vi "FFT.vi"() -> ()   [LabVIEW 2021]
uses:
  ark_all/arkady-arxiv/cursor winow sygnal plot.ctl
  ark_all/arkady-arxiv/show-win- control.ctl
  ark_all/arkady-arxiv/cursor window action.ctl
  <vilib>/measure/maspectr.llb/FFT Power Spectrum for N Chan.vi
  <vilib>/measure/NI_MAPro.lvlib
panel:
  out "time (sec)":dbl=0.04508427
  in  "offset factor":dbl=100.0
  out "win (sec)":dbl=0.010354
  in  "digitization freq":dbl=3000000.0
  in  "win 2":T1={"cen (Hz)"=32754.180483243686, "win (Hz)"=308.86311527720136, "left (Hz)"=32599.748925605087, "right (Hz)"=32908.61204088229} {"right (Hz)" format="%#_3p"}
  out "dt (sec)":dbl=3.3e-07
  in  "cursor window":T2={"left"=0.04139793333333315, "right "=0.05175193333333315, "center"=0.04657493333333315, "window"=0.010354, "cursors"=[0, 1, 2], "relative"=0, "absolute"=0, "fixed vertical offset"=0.0, "vertical offset"=0.0, "skew"=0.0, "default window frac"=0.1, "kind"=enum."symmetric", "skew.left"=0.5, "skew.right"=0.5, "wing order"=enum."back", "Plot ref Syg"=refnum}
  in  "run":bool
  in  "Data window":T3={"Start"=124194, "Length"=31062, "Channel numbers"=[0], "Cannel names"=["freq", ""], "Group name"="p"}
  out "Signal graph":waveform(dbl)[](graph)=[{"t0"=timestamp(-0.009969989999999984 s since 1904-01-01), "dt"=3.3e-07, "Y"=array[333333 elements], "attributes"=variant("Configuration"=variant(string "[Configuration]\nConfiguration.Post-trigger delay = \"-0.010000000000\"\nConfiguration.Post-trigger duration = \"0.10000000000\"\nConfiguration.Rate = \"3030303.0303\"\nConfiguration.Ranges = \"<size(s)=5> 10.000000000 10.000000000 10.000000000 1.0000000000 1.0000000000\"\nConfiguration.Re-name channels.<size(s)> = \"5\"\nConfiguration.Re-name channels 0 = \"Idot\"\nConfiguration.Re-name channels 1 = \"Bdot\"\nConfiguration.Re-name channels 2 = \"Bproj\"\nConfiguration.Re-name channels 3 = \"freq\"\nConfiguration.Re-name channels 4 = \"drive\"\nConfiguration.Active channels = \"0,1,2,5,6\"\nConfiguration.External\\nclock = \"FALSE\"\nConfiguration.Monitor time\\nconstant = \"1.0000000000\"\nConfiguration.Sync = \"TRUE\"\nConfiguration.Lock-in input channel phases = \"<size(s)=0> \"\nConfiguration.Output channels configuration.<size(s)> = \"0\""), "NI_ChannelName"=variant(string "freq"))}]
  in  "Preserve old data":bool=TRUE
  out "FFT Graph":cluster{"f0":dbl, "df":dbl, "magnitude":dbl[]}[](graph)=[{"f0"=0.0, "df"=97.55659746001642, "magnitude"=array[15531 elements]}, {"f0"=0.0, "df"=97.55659746001642, "magnitude"=array[15531 elements]}, {"f0"=0.0, "df"=97.55659746001642, "magnitude"=array[15531 elements]}, {"f0"=0.0, "df"=97.55659746001642, "magnitude"=array[15531 elements]}, {"f0"=0.0, "df"=97.55659746001642, "magnitude"=array[15531 elements]}, {"f0"=0.0, "df"=97.55659746001642, "magnitude"=array[15531 elements]}, {"f0"=0.0, "df"=97.55659746001642, "magnitude"=array[15531 elements]}, {"f0"=0.0, "df"=97.55659746001642, "magnitude"=array[15531 elements]}, {"f0"=0.0, "df"=97.55659746001642, "magnitude"=array[15531 elements]}, {"f0"=0.0, "df"=97.55659746001642, "magnitude"=array[15531 elements]}, {"f0"=0.0, "df"=97.55659746001642, "magnitude"=array[15531 elements]}, {"f0"=0.0, "df"=97.55659746001642, "magnitude"=array[15531 elements]}, {"f0"=0.0, "df"=97.55659746001642, "magnitude"=array[15531 elements]}, {"f0"=0.0, "df"=97.55659746001642, "magnitude"=array[15531 elements]}, {"f0"=0.0, "df"=97.55659746001642, "magnitude"=array[15531 elements]}, {"f0"=0.0, "df"=97.55659746001642, "magnitude"=array[15531 elements]}, {"f0"=0.0, "df"=97.55659746001642, "magnitude"=array[15531 elements]}, {"f0"=0.0, "df"=97.55659746001642, "magnitude"=array[15531 elements]}, {"f0"=0.0, "df"=97.55659746001642, "magnitude"=array[15531 elements]}, {"f0"=0.0, "df"=97.55659746001642, "magnitude"=array[15531 elements]}, {"f0"=0.0, "df"=97.55659746001642, "magnitude"=array[15531 elements]}, {"f0"=0.0, "df"=97.55659746001642, "magnitude"=array[15531 elements]}, {"f0"=0.0, "df"=97.55659746001642, "magnitude"=array[15531 elements]}, {"f0"=0.0, "df"=97.55659746001642, "magnitude"=array[15531 elements]}, {"f0"=0.0, "df"=97.55659746001642, "magnitude"=array[15531 elements]}, {"f0"=0.0, "df"=97.55659746001642, "magnitude"=array[15531 elements]}, {"f0"=0.0, "df"=97.55659746001642, "magnitude"=array[15531 elements]}, {"f0"=0.0, "df"=97.55659746001642, "magnitude"=array[15531 elements]}, {"f0"=0.0, "df"=97.55659746001642, "magnitude"=array[15531 elements]}, {"f0"=0.0, "df"=97.55659746001642, "magnitude"=array[15531 elements]}, {"f0"=0.0, "df"=97.55659746001642, "magnitude"=array[15531 elements]}, {"f0"=0.0, "df"=97.55659746001642, "magnitude"=array[15531 elements]}, {"f0"=0.0, "df"=97.55659746001642, "magnitude"=array[15531 elements]}, {"f0"=0.0, "df"=97.55659746001642, "magnitude"=array[15531 elements]}, {"f0"=0.0, "df"=97.55659746001642, "magnitude"=array[15531 elements]}, {"f0"=0.0, "df"=97.55659746001642, "magnitude"=array[15531 elements]}, {"f0"=0.0, "df"=97.55659746001642, "magnitude"=array[15531 elements]}, {"f0"=0.0, "df"=97.55659746001642, "magnitude"=array[15531 elements]}, {"f0"=0.0, "df"=97.55659746001642, "magnitude"=array[15531 elements]}, {"f0"=0.0, "df"=97.55659746001642, "magnitude"=array[15531 elements]}, {"f0"=0.0, "df"=97.55659746001642, "magnitude"=array[15531 elements]}, {"f0"=0.0, "df"=97.55659746001642, "magnitude"=array[15531 elements]}, {"f0"=0.0, "df"=97.55659746001642, "magnitude"=array[15531 elements]}, {"f0"=0.0, "df"=97.55659746001642, "magnitude"=array[15531 elements]}, {"f0"=0.0, "df"=97.55659746001642, "magnitude"=array[15531 elements]}, {"f0"=0.0, "df"=97.55659746001642, "magnitude"=array[15531 elements]}, {"f0"=0.0, "df"=97.55659746001642, "magnitude"=array[15531 elements]}, {"f0"=0.0, "df"=97.55659746001642, "magnitude"=array[15531 elements]}, {"f0"=0.0, "df"=97.55659746001642, "magnitude"=array[15531 elements]}, {"f0"=0.0, "df"=97.55659746001642, "magnitude"=array[15531 elements]}, {"f0"=0.0, "df"=97.55659746001642, "magnitude"=array[15531 elements]}, {"f0"=0.0, "df"=97.55659746001642, "magnitude"=array[15531 elements]}, {"f0"=0.0, "df"=97.55659746001642, "magnitude"=array[15531 elements]}, {"f0"=0.0, "df"=97.55659746001642, "magnitude"=array[15531 elements]}, {"f0"=0.0, "df"=97.55659746001642, "magnitude"=array[15531 elements]}]
  in  "Data File Type":T4(ring)
  in  "Window":u32(ring)=1 items=["Rectangle"=0, "Hanning"=1, "Hamming"=2, "Blackman-Harris"=3, "Exact Blackman"=4, "Blackman"=5, "Flat Top"=6, "4 Term B-Harris "=7, "7 Term B-Harris"=8, "Low Sidelobe"=9, "Blackman Nuttall"=11, "Triangle"=30, "Bartlett-Hanning"=31, "Bohman"=32, "Parzen"=33, "Welch"=34, "Kaiser"=60, "Dolph-Chebyshev"=61, "Gaussian"=62]
  in  "Input file path":path=path "/Users/arkady/Desktop/shared__vikram_shiva_zoltan--Aug2025/August_2025/082225/p_c4_019_082225.tdms"
  # "OR"
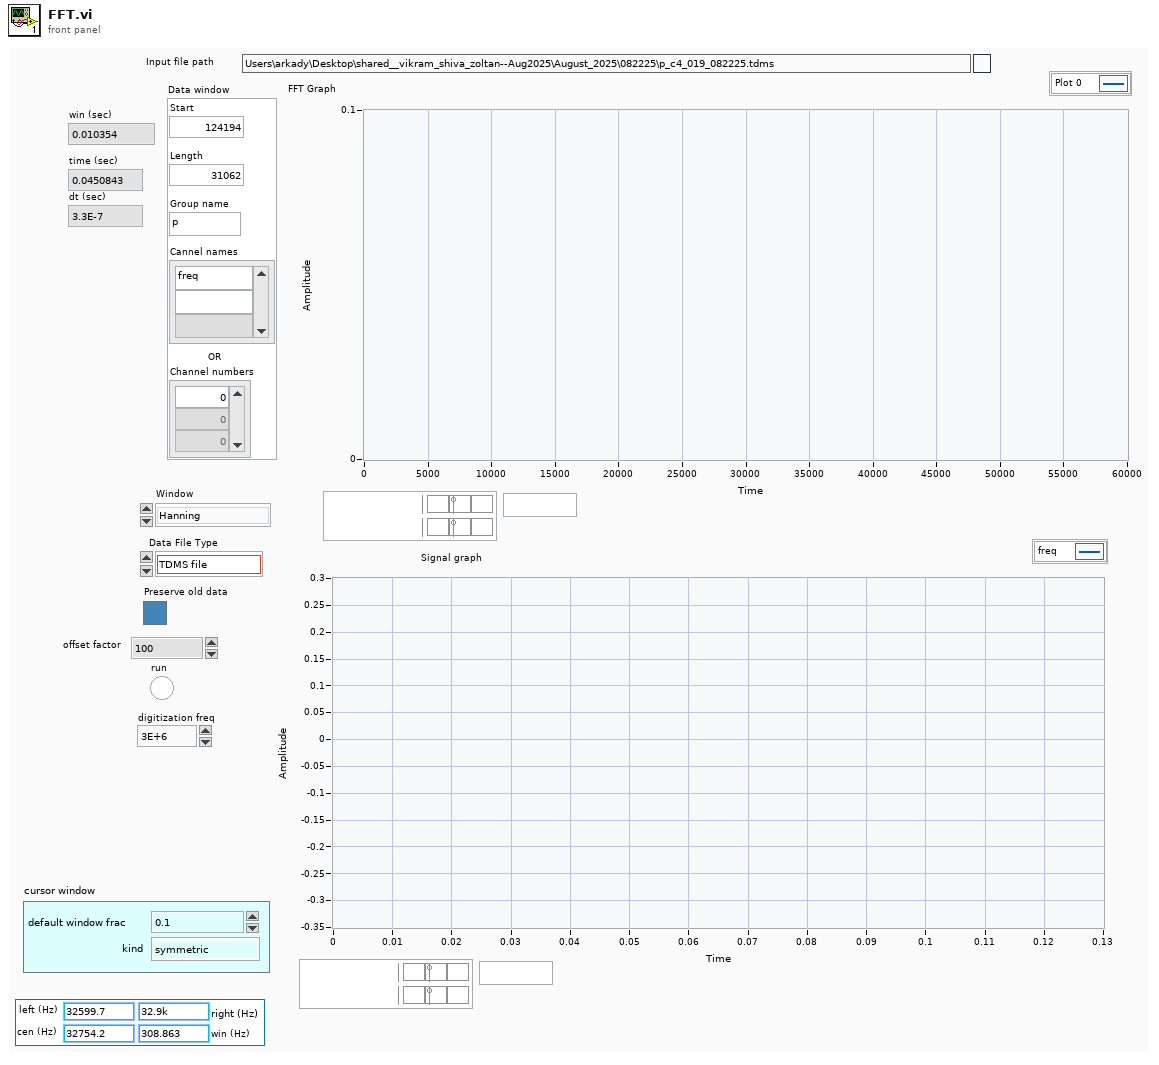
[diagram p1: front panel]
types:
  T1 = typedef "show-win- control.ctl" = cluster{"cen (Hz)":dbl, "win (Hz)":dbl, "left (Hz)":dbl, "right (Hz)":dbl}
  T2 = typedef "cursor winow sygnal plot.ctl" = cluster{"left":dbl, "right ":dbl, "center":dbl, "window":dbl, "cursors":i32[], "relative":i32, "absolute":i32, "fixed vertical offset":dbl, "vertical offset":dbl, "skew":dbl, "default window frac":dbl, "kind":enum16{"symmetric", "skewed", "fancy"}, "skew.left":dbl, "skew.right":dbl, "wing order":enum16{"forw", "back"}, "Plot ref Syg":refnum<vi>}
  T3 = cluster{"Start":i64, "Length":i32, "Channel numbers":i64[], "Cannel names":string[], "Group name":string}
  T4 = enum16{"TDMS file", "Tektronics ISF", "BinF file", "ASCII File", "BinH File", "BinW File", "BINARY File"}
  T5 = typedef "cursor window action.ctl" = enum16{"balance", "h. offset change", "cursor moves", "change center", "change window", "init", "check", "reset", "set y to middle", "idle", "-write all Y", "-write left.X", "-write center.X", "-write right.X", "-write all X", "-change center", "-change window", "-change skew", "-read cursor 2", "-read cursor 1", "-read cursor 0", "-read all cursors", "-reset", "-read plot scale", "-set y to middle", "-Q: center.Y is visible", "-Q: window is visible", "-parse center.Y", "-right left from center", "-left move", "-right move", "-set center.Y", "-empty", "-set cursors to default", "-check", "-write center.Y", "-copy cursor 1", "-copy cursor 0", "-copy cursor 2", "move right", "move left", "shrink", "broaden", "skew up", "skew down", "-write plot scale", "zoom X", "change cen&win", "zoom to all data", "color--red", "color--green", "color--yellow", "read", "zoom out", "zoom in", "slide right", "slide left", "set range aspect ratio to 1", "move to window range", "--move to window range"}
  T6 = typedef "eventvkey.ctl" = enum16{"ASCII", "Enter", "Return", "Shift", "Ctrl", "Alt", "Cmd", "Opt", "Caps", "NumLock", "Clear", "Break", "Up", "Down", "Left", "Right", "Insert", "Delete", "Home", "End", "PageUp", "PageDown", "Escape", "Help", "Pause", "ScrollLock", "F1", "F2", "F3", "F4", "F5", "F6", "F7", "F8", "F9", "F10", "F11", "F12", "F13", "F14", "F15", "F16", "F17", "F18", "F19", "F20", "F21", "F22", "F23", "F24", "Play", "VolumeUp", "VolumeDown", "Mute", "Two Byte Char"}
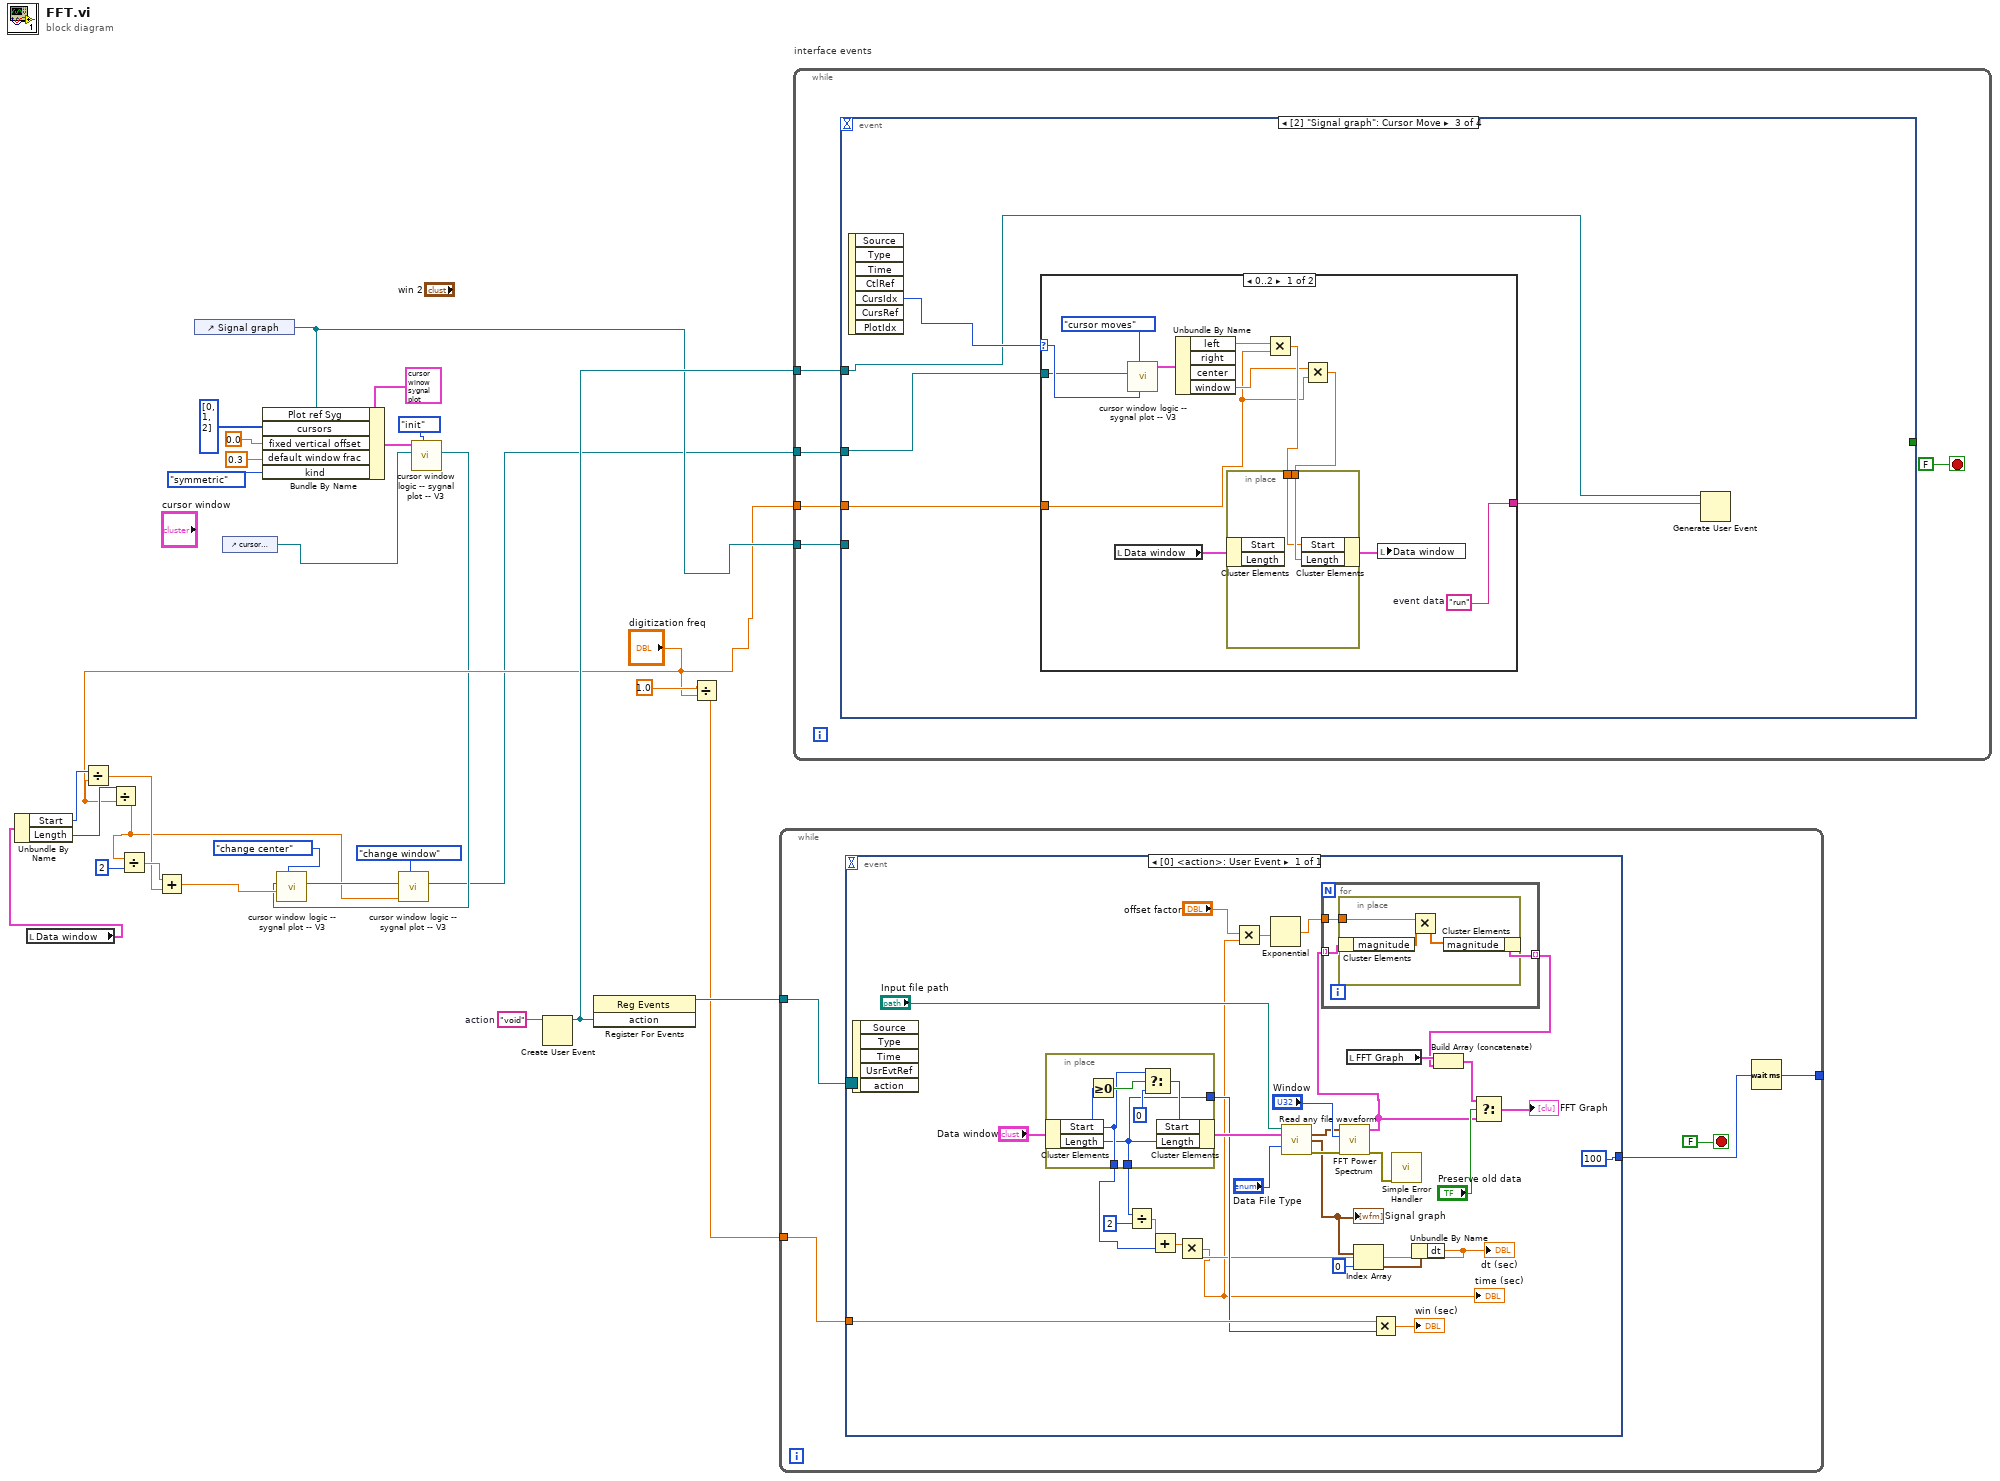
[diagram p0: block diagram]
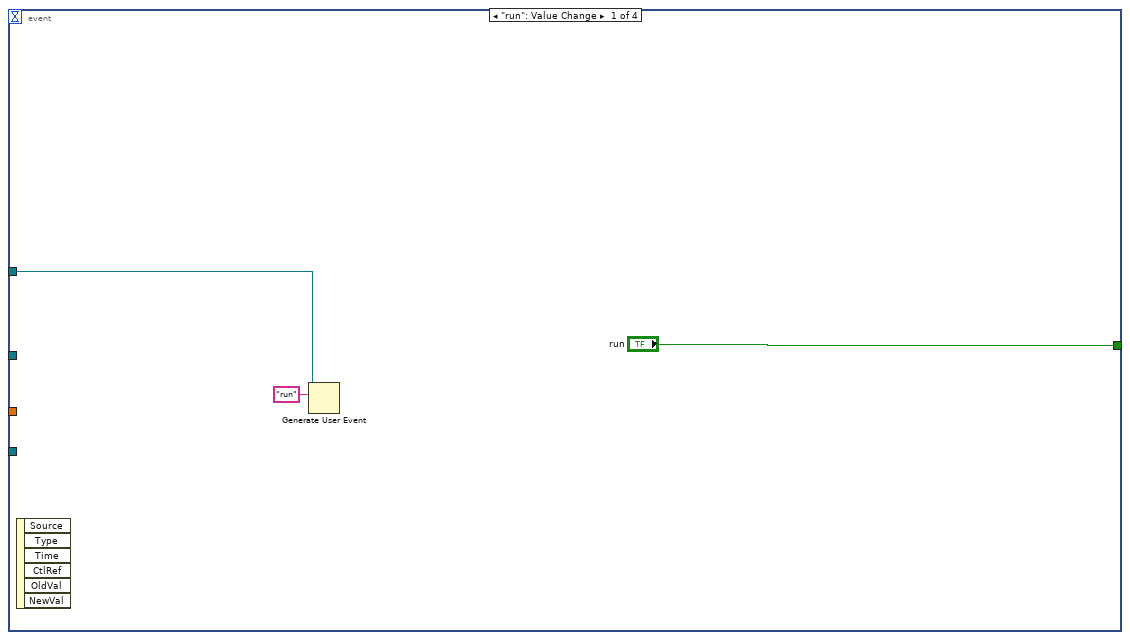
[diagram p2: hidden frame]
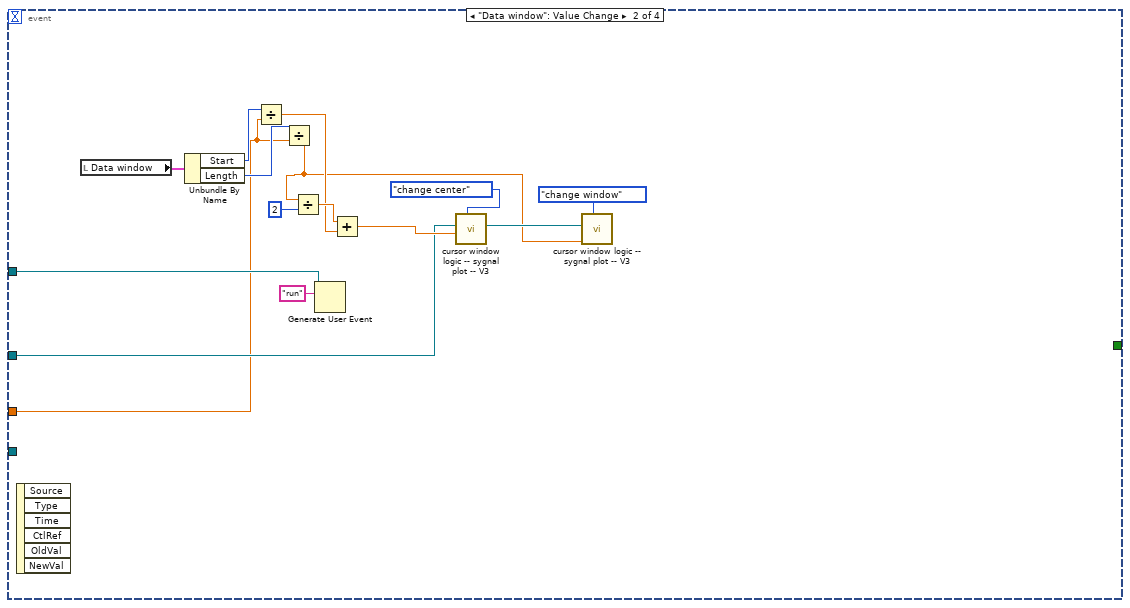
[diagram p3: hidden frame]
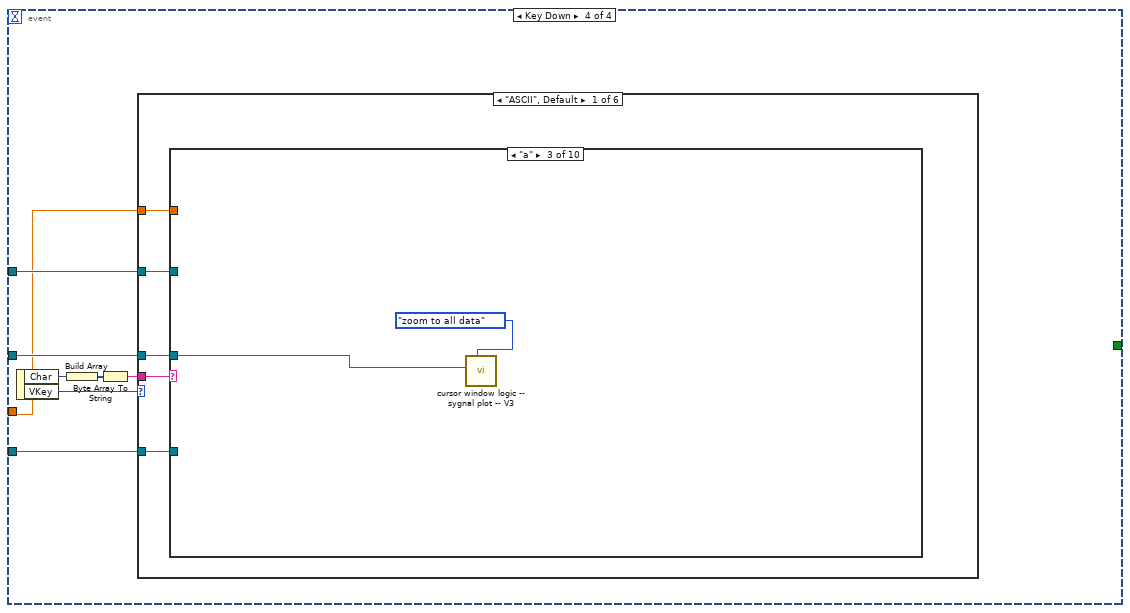
[diagram p5: hidden frame]
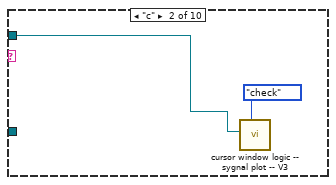
[diagram p7: hidden frame]
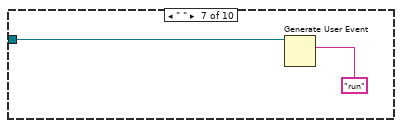
[diagram p11: hidden frame]
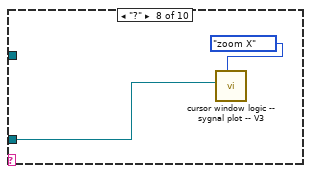
[diagram p12: hidden frame]
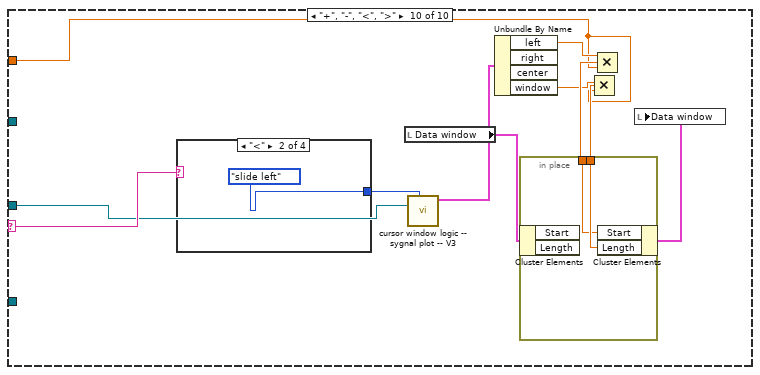
[diagram p14: hidden frame]
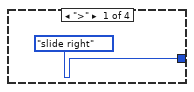
[diagram p15: hidden frame]
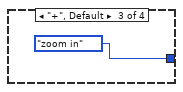
[diagram p16: hidden frame]
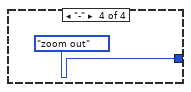
[diagram p17: hidden frame]
diagram:
  w28 = "void"  # action
  n1 = local read "Data window"() -> (w4:T3)
  n2 = Unbundle By Name(w4) -> ("Start"=w5:i64, "Length"=w8:i32)
  n3 = Divide(x=w5, y="digitization freq") -> (x/y=w7:dbl)
  n4 = Divide(x=w8, y="digitization freq") -> (x/y=w6:dbl)
  n5 = Divide(x=w6, y=2) -> (x/y=w10:dbl)
  n6 = Add(x=w10, y=w7) -> (x+y=w9:dbl)
  n7 = control-ref of="Signal graph"() -> (w17:refnum<vi>)
  n8 = control-ref of="cursor window"() -> (w18:refnum<vi>)
  n9 = Bundle By Name(cluster=T2 {"left"=2378.60310421286, "right "=2421.6740576496672, "center"=2421.6740576496672, "window"=2421.6740576496672, "cursors"=[], "relative"=0, "absolute"=0, "fixed vertical offset"=2421.6740576496672, "vertical offset"=2421.6740576496672, "skew"=2421.6740576496672, "default window frac"=2421.6740576496672, "kind"=enum."skewed", "skew.left"=2421.6740576496672, "skew.right"=2421.6740576496672, "wing order"=enum."back", "Plot ref Syg"=refnum} ("cursor bracket: All, data window"), "Plot ref Syg"=w17, "cursors"=i32[] [0, 1, 2], "fixed vertical offset"=0.0, "default window frac"=0.3 ("fixed vertical offset"), "kind"=enum16{"symmetric", "skewed", "fancy"}."symmetric") -> (w21:T2)
  n10 = call "cursor window logic -- sygnal plot -- V3.vi"("cursor window action"=cursor_window_action."init", "cursor window IN"=w18, "cursor window init"=w21) -> ("cursor window OUT"=w2:refnum<vi>)  [unwired: 7 in, 1 out]
  n11 = call "cursor window logic -- sygnal plot -- V3.vi"("cursor window action"=cursor_window_action."change center", "center"=w9, "cursor window IN"=w2) -> ("cursor window OUT"=w12:refnum<vi>)  [unwired: 7 in, 1 out]
  n12 = call "cursor window logic -- sygnal plot -- V3.vi"("cursor window action"=cursor_window_action."change window", "window"=w6, "cursor window IN"=w12) -> ("cursor window OUT"=w1:refnum<vi>)  [unwired: 7 in, 1 out]
  n13 = Create User Event(user event datatype=w28) -> (user event=w26:refnum<user-event>)  [unwired: 1 in, 1 out]
  n14 = register-events(w26) -> (reference out=w27:refnum<event-registration>)  [unwired: 2 in, 1 out]
  n15 = Divide(x=1.0, y="digitization freq") -> (x/y=w15:dbl)
  n16 = while {
    tunnel: w27 -> [w32]
    tunnel: [w31] -> _
    tunnel: w15 -> [w29]
    stop <- FALSE stop-if-true
    n17 = event shown="[0] <action>: User Event" {
      selector: w32 -> [_]
      dyn-events: _ -> [_]
      timeout: _ -> [_]
      tunnel: [u32 100 ("milliseconds to wait")] -> w30
      tunnel: w29 -> [w48]
      event User Event {
        n18 = event-data() -> ()  [unwired: 1 in, 5 out]
        n19 = in-place {
          in-place-border: [w71] -> w47
          in-place-border: [w72] -> w40
          in-place-border: [w71] -> w43
          n20 = in-place-cluster #1("Data window") -> ("Start"=w72:i64, "Length"=w71:i32)
          n21 = Greater Or Equal To 0?(x=w72) -> (x >= 0?=w75:bool)
          n22 = Select(t=w72, s=w75, f=i64 0 ("Start")) -> (s? t:f=w74:i64)
          n23 = in-place-cluster #1("Start"=w74, "Length"=w71) -> (w50:T3)
        }
        n24 = Divide(x=w43, y=2) -> (x/y=w41:dbl)
        n25 = Add(x=w41, y=w40) -> (x+y=w39:dbl)
        n26 = call "Read any file waveform.vi"("Input file path"="Input file path", "Data window"=w50, "Data File Type"="Data File Type") -> ("Data out"=w54:waveform(dbl)[], "All Data out"=w49:waveform(dbl)[], "error out"=w63:errorcluster)  [unwired: 7 in, 3 out]
        "Signal graph" <- w49
        n27 = call-poly <vilib>:"FFT Power Spectrum.vi"("error in (no error)"=w63, "window"="Window", "time signals"=w54) -> ("error out"=w56:errorcluster, "power spectra"=w45:cluster{"f0":dbl, "df":dbl, "magnitude":dbl[]}[])  [unwired: 3 in, 4 out]
        n28 = local read "FFT Graph"() -> (w61:cluster{"f0":dbl, "df":dbl, "magnitude":dbl[]}[])
        n29 = Index Array(array=w49, index=0) -> (element=w52:waveform(dbl))
        n30 = Multiply(x=w48, y=w47) -> (x*y=→"win (sec)":dbl)
        n31 = call <vilib>:"Simple Error Handler.vi"("error in (no error)"=w56) -> ()  [unwired: 4 in, 5 out]
        n32 = Unbundle By Name(w52) -> ("dt"=w38:dbl)
        "dt (sec)" <- w38
        n33 = Multiply(x=w39, y=w38) -> (x*y=w36:dbl)
        "time (sec)" <- w36
        n34 = Multiply(x="offset factor", y=w36) -> (x*y=w35:dbl)
        n35 = Exponential(1:w35) -> (0:w34:dbl)
        n36 = for {
          tunnel: w45 -> [w67] mode=indexing
          tunnel: [w66] -> w44 mode=indexing
          tunnel: w34 -> [w65]
          n37 = in-place {
            in-place-border: w65 -> [w69]
            n38 = in-place-cluster #2(w67) -> ("magnitude"=w70:dbl[])
            n39 = Multiply(x=w69, y=w70) -> (x*y=w68:dbl[])
            n40 = in-place-cluster #2("magnitude"=w68) -> (w66:cluster{"f0":dbl, "df":dbl, "magnitude":dbl[]})
          }
        }
        n41 = Build Array (concatenate)(w61, w44) -> (w60:cluster{"f0":dbl, "df":dbl, "magnitude":dbl[]}[])
        n42 = Select(t=w60, s="Preserve old data", f=w45) -> (s? t:f=→"FFT Graph":cluster{"f0":dbl, "df":dbl, "magnitude":dbl[]}[])
      }
    }
    n43 = Wait (ms)(milliseconds to wait=w30) -> (millisecond timer value=w31:u32)
  }
  n44 = while "interface events" {
    tunnel: w26 -> [w79]
    tunnel: w17 -> [w78]
    tunnel: w1 -> [w77]
    tunnel: "digitization freq" -> [w76]
    stop <- FALSE stop-if-true
    n45 = event shown="[2] \"Signal graph\": Cursor Move" {
      selector: _ -> [_ _ _ _]
      dyn-events: _ -> [_ _ _ _]
      timeout: _ -> [_ _ _ _]
      tunnel: ["run" _ _ _] -> _
      tunnel: w79 -> [w82 w98 w100 w121]
      tunnel: w78 -> [_ _ _ w120]
      tunnel: w77 -> [_ w89 w102 w119]
      tunnel: w76 -> [_ w84 w99 w118]
      event "run": Value Change {
        n46 = event-data() -> ()  [unwired: 1 in, 6 out]
        n47 = Generate User Event(user event=w82, event data cluster="run" ("event data")) -> ()  [unwired: 2 in, 2 out]
      }
      event "Data window": Value Change {
        n48 = event-data() -> ()  [unwired: 1 in, 6 out]
        n49 = local read "Data window"() -> (w93:T3)
        n50 = Unbundle By Name(w93) -> ("Start"=w85:i64, "Length"=w88:i32)
        n51 = Divide(x=w85, y=w84) -> (x/y=w87:dbl)
        n52 = Divide(x=w88, y=w84) -> (x/y=w86:dbl)
        n53 = Divide(x=w86, y=2) -> (x/y=w91:dbl)
        n54 = Generate User Event(user event=w98, event data cluster="run" ("event data")) -> ()  [unwired: 2 in, 2 out]
        n55 = Add(x=w91, y=w87) -> (x+y=w90:dbl)
        n56 = call "cursor window logic -- sygnal plot -- V3.vi"("cursor window action"=cursor_window_action."change center", "center"=w90, "cursor window IN"=w89) -> ("cursor window OUT"=w94:refnum<vi>)  [unwired: 7 in, 1 out]
        n57 = call "cursor window logic -- sygnal plot -- V3.vi"("cursor window action"=cursor_window_action."change window", "window"=w86, "cursor window IN"=w94) -> ()  [unwired: 7 in, 2 out]
      }
      event "Signal graph": Cursor Move {
        n58 = event-data() -> ("CursIdx"=w103:i32)  [unwired: 1 in, 6 out]
        n59 = case shown="0..2" w103 {
          selector: w103 -> [w114 _]
          tunnel: w102 -> [w112 _]
          tunnel: [w109 _] -> w101
          tunnel: w99 -> [w105 _]
          frame 0..2 {
            w109 = "run"  # event data
            n60 = local read "Data window"() -> (w111:T3)
            n61 = call "cursor window logic -- sygnal plot -- V3.vi"("CursIdx"=w114, "cursor window action"=cursor_window_action."cursor moves", "cursor window IN"=w112) -> ("cursor window out"=w113:T2)  [unwired: 7 in, 1 out]
            n62 = Unbundle By Name(w113) -> ("left"=w108:dbl, "window"=w106:dbl)  [unwired: 2 out]
            n63 = Multiply(x=w108, y=w105) -> (x*y=w107:dbl)
            n64 = Multiply(x=w106, y=w105) -> (x*y=w104:dbl)
            n65 = in-place {
              in-place-border: w104 -> [w117]
              in-place-border: w107 -> [w116]
              n66 = in-place-cluster #3(w111) -> ()  [unwired: 2 out]
              n67 = in-place-cluster #3("Start"=w116, "Length"=w117) -> (w110:T3)
            }
            n68 = local write "Data window"(w110) -> ()
          }
          frame 3, Default {
          }
        }
        n69 = Generate User Event(user event=w100, event data cluster=w101) -> ()  [unwired: 2 in, 2 out]
      }
      event Key Down {
        n70 = event-data() -> ("Char"=w123:i16, "VKey"=w125:T6)  [unwired: 1 in]
        n71 = Build Array(w123) -> (w124:i16[])
        n72 = Byte Array To String(unsigned byte array=w124) -> (string=w122:string)
        n73 = case shown="\"ASCII\", Default" w125 {
          selector: w125 -> [_ _ _ _ _ w168]
          tunnel: w122 -> [w130 _ _ _ _ _]
          tunnel: w121 -> [w129 _ _ _ _ w156]
          tunnel: w120 -> [w128 _ _ _ _ _]
          tunnel: w119 -> [w127 _ _ _ _ w167]
          tunnel: w118 -> [w126 _ _ _ _ w160]
          frame "ASCII", Default {
            n74 = case shown="\"a\"" w130 {
              selector: w130 -> [_ _ _ _ _ _ _ _ _ w148]
              tunnel: w129 -> [_ _ _ _ _ _ w135 _ _ _]
              tunnel: w128 -> [_ _ _ _ _ _ _ _ _ _]
              tunnel: w127 -> [_ w131 w133 _ _ _ _ w137 _ w147]
              tunnel: w126 -> [_ _ _ _ _ _ _ _ _ w139]
              frame "0", Default {
              }
              frame "c" {
                n75 = call "cursor window logic -- sygnal plot -- V3.vi"("cursor window action"=cursor_window_action."check", "cursor window IN"=w131) -> ()  [unwired: 8 in, 2 out]
              }
              frame "a" {
                n76 = call "cursor window logic -- sygnal plot -- V3.vi"("cursor window action"=cursor_window_action."zoom to all data", "cursor window IN"=w133) -> ()  [unwired: 8 in, 2 out]
              }
              frame "s" {
              }
              frame "~" {
              }
              frame "l" {
              }
              frame " " {
                n77 = Generate User Event(user event=w135, event data cluster="run" ("event data")) -> ()  [unwired: 2 in, 2 out]
              }
              frame "?" {
                n78 = call "cursor window logic -- sygnal plot -- V3.vi"("cursor window action"=cursor_window_action."zoom X", "cursor window IN"=w137) -> ()  [unwired: 8 in, 2 out]
              }
              frame ",", "." {
              }
              frame "+", "-", "<", ">" {
                n79 = case shown="\"<\"" w148 {
                  tunnel: [cursor_window_action."slide right" ("cursor window action") cursor_window_action."slide left" ("cursor window action") cursor_window_action."zoom in" ("cursor window action") cursor_window_action."zoom out" ("cursor window action")] -> w149
                  frame ">" {
                  }
                  frame "<" {
                  }
                  frame "+", Default {
                  }
                  frame "-" {
                  }
                }
                n80 = local read "Data window"() -> (w145:T3)
                n81 = call "cursor window logic -- sygnal plot -- V3.vi"("cursor window action"=w149, "cursor window IN"=w147) -> ("cursor window out"=w144:T2)  [unwired: 8 in, 1 out]
                n82 = Unbundle By Name(w144) -> ("left"=w143:dbl, "window"=w141:dbl)  [unwired: 2 out]
                n83 = Multiply(x=w141, y=w139) -> (x*y=w140:dbl)
                n84 = Multiply(x=w143, y=w139) -> (x*y=w142:dbl)
                n85 = in-place {
                  in-place-border: w140 -> [w151]
                  in-place-border: w142 -> [w150]
                  n86 = in-place-cluster #4(w145) -> ()  [unwired: 2 out]
                  n87 = in-place-cluster #4("Start"=w150, "Length"=w151) -> (w146:T3)
                }
                n88 = local write "Data window"(w146) -> ()
              }
            }
          }
          frame "PageUp" {
          }
          frame "Enter" {
          }
          frame "Caps" {
          }
          frame "PageDown" {
          }
          frame "Up".."Right" {
            n89 = case shown="\"Right\"" w168 {
              tunnel: [cursor_window_action."broaden" ("cursor window action") cursor_window_action."shrink" ("cursor window action") cursor_window_action."move left" ("cursor window action") cursor_window_action."move right" ("cursor window action")] -> w166
              frame "Up", Default {
              }
              frame "Down" {
              }
              frame "Left" {
              }
              frame "Right" {
              }
            }
            n90 = local read "Data window"() -> (w163:T3)
            n91 = call "cursor window logic -- sygnal plot -- V3.vi"("cursor window action"=w166, "cursor window IN"=w167) -> ("cursor window out"=w165:T2)  [unwired: 8 in, 1 out]
            n92 = Unbundle By Name(w165) -> ("left"=w162:dbl, "window"=w161:dbl)  [unwired: 2 out]
            n93 = Multiply(x=w161, y=w160) -> (x*y=w159:dbl)
            n94 = Multiply(x=w162, y=w160) -> (x*y=w158:dbl)
            n95 = in-place {
              in-place-border: w159 -> [w170]
              in-place-border: w158 -> [w169]
              n96 = in-place-cluster #5(w163) -> ()  [unwired: 2 out]
              n97 = in-place-cluster #5("Start"=w169, "Length"=w170) -> (w164:T3)
            }
            n98 = local write "Data window"(w164) -> ()
            n99 = Generate User Event(user event=w156, event data cluster="run" ("event data")) -> ()  [unwired: 2 in, 2 out]
          }
        }
      }
    }
  }
